vi "gyro-V5.vi"() -> ()   [LabVIEW 2017] (continued)
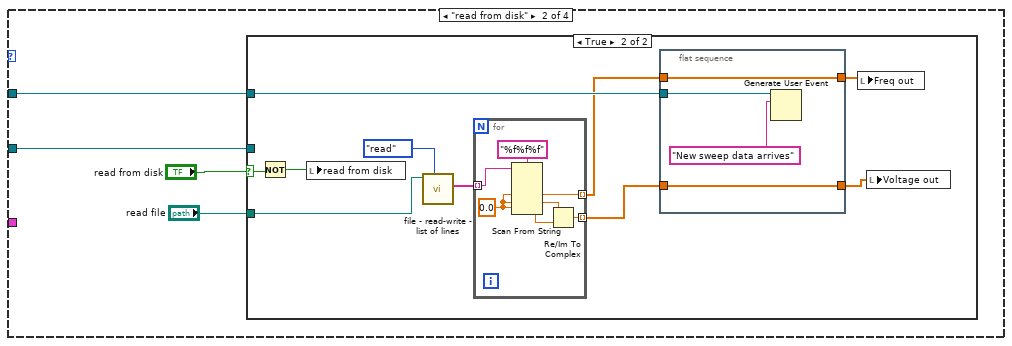
[diagram p4: hidden frame]
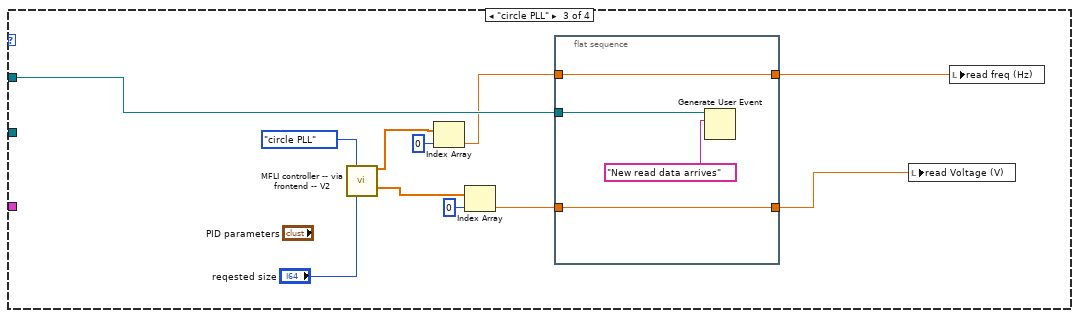
[diagram p6: hidden frame]
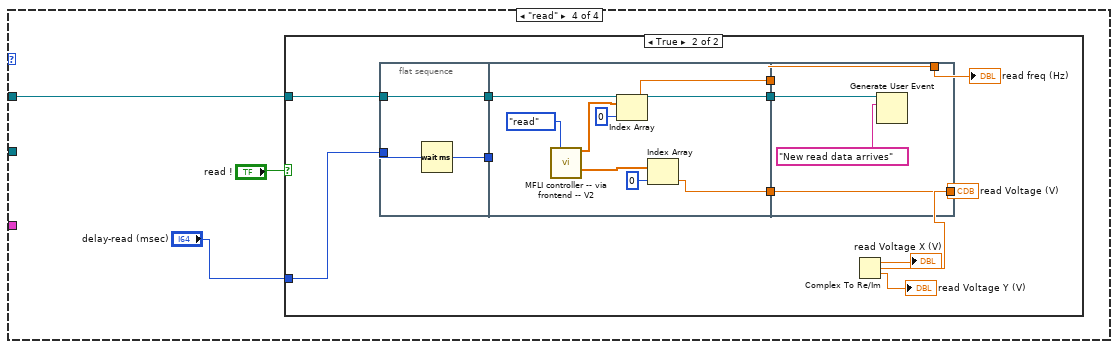
[diagram p7: hidden frame]
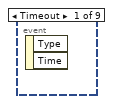
[diagram p9: hidden frame]
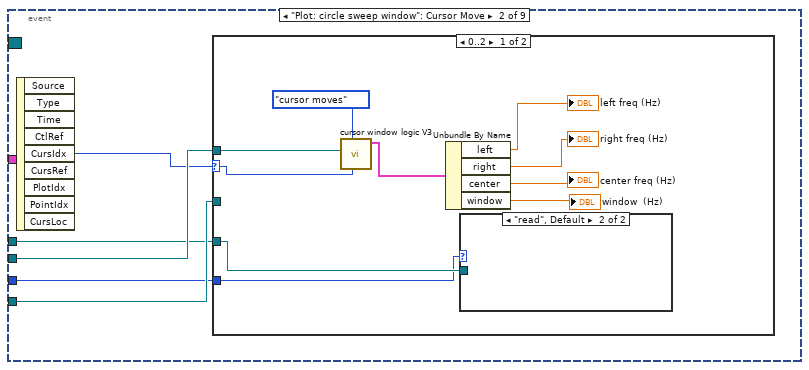
[diagram p10: hidden frame]
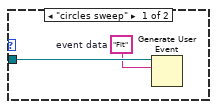
[diagram p11: hidden frame]
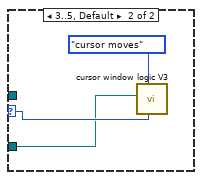
[diagram p12: hidden frame]
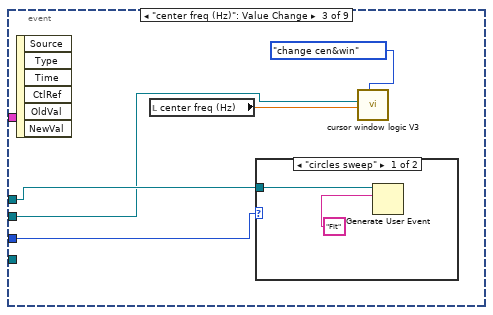
[diagram p13: hidden frame]
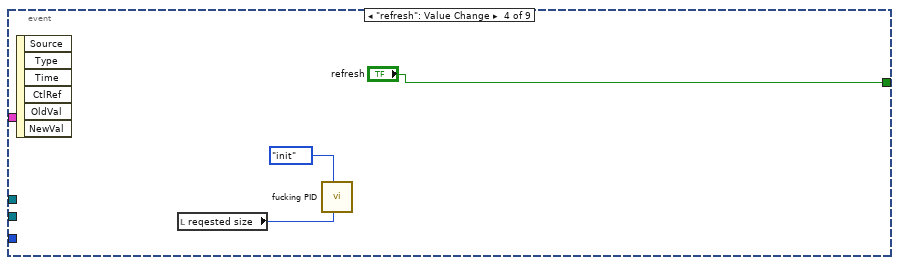
[diagram p15: hidden frame]
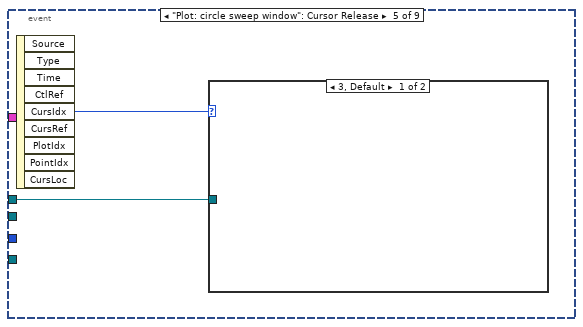
[diagram p16: hidden frame]
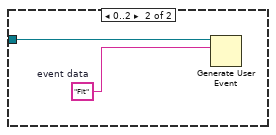
[diagram p17: hidden frame]
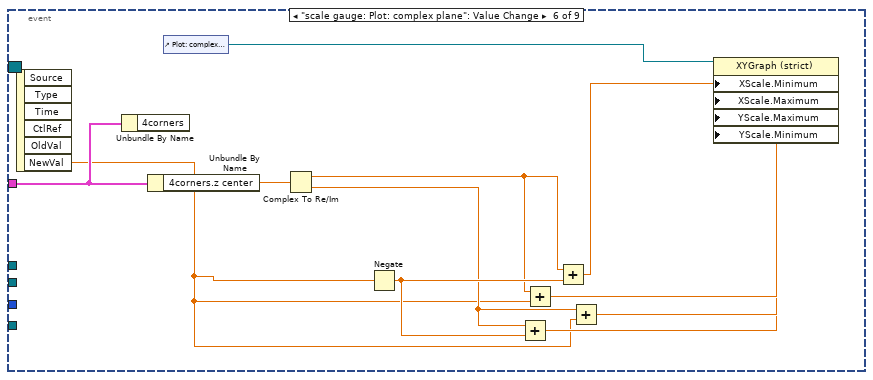
[diagram p18: hidden frame]
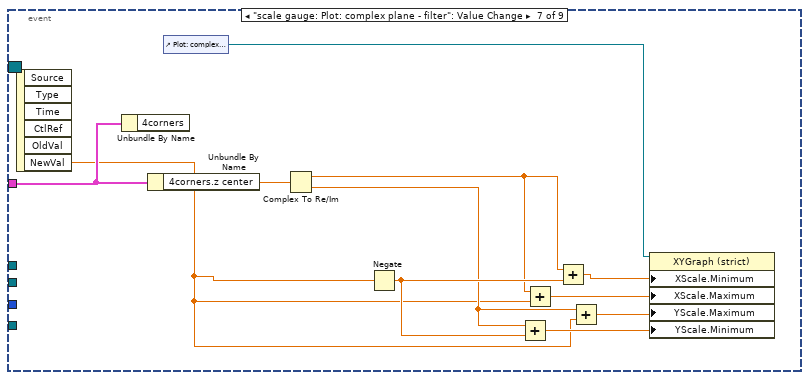
[diagram p19: hidden frame]
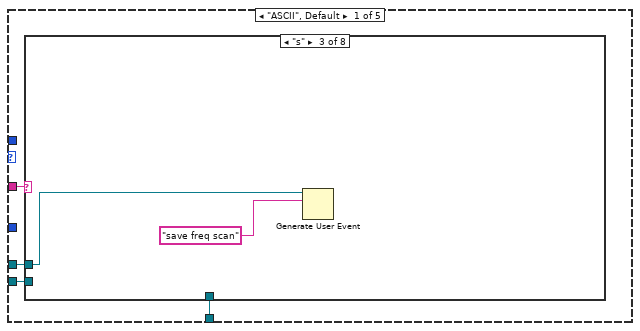
[diagram p20: hidden frame]
                  n39 = Re/Im To Complex(1:w95, 2:w96) -> (0:w94:cdb)
                }
                n40 = flat-sequence {
                  tunnel: w86 -> [w103]
                  tunnel: [w103] -> w85
                  tunnel: w92 -> [w102]
                  tunnel: [w101] -> w84
                  tunnel: w83 -> [w101]
                  frame #0 {
                    n41 = Generate User Event(user event=w102, event data cluster="New sweep data arrives" ("event data")) -> ()  [unwired: 2 in, 2 out]
                  }
                }
                n42 = local write "Freq out"(w85) -> ()
                n43 = local write "Voltage out"(w84) -> ()
              }
            }
          }
          frame "circle PLL" {
            n44 = call "MFLI controller -- via frontend -- V2.vi"("MFLI controller action"=MFLI_controller_action."circle PLL", "reqested size"="reqested size") -> ("Freq out (Hz)"=w111:dbl[], "Voltage out (V)"=w110:cdb[])  [unwired: 11 in, 1 out]
            n45 = Index Array(array=w111, index=0) -> (element=w107:dbl)
            n46 = Index Array(array=w110, index=0) -> (element=w105:cdb)
            n47 = flat-sequence {
              tunnel: w109 -> [w117]
              tunnel: [w116] -> w108
              tunnel: w107 -> [w116]
              tunnel: [w115] -> w106
              tunnel: w105 -> [w115]
              frame #0 {
                n48 = Generate User Event(user event=w117, event data cluster="New read data arrives" ("event data")) -> ()  [unwired: 2 in, 2 out]
              }
            }
            n49 = local write "read Voltage (V)"(w106) -> ()
            n50 = local write "read freq (Hz)"(w108) -> ()
          }
          frame "read" {
            n51 = case shown="True" "read !" {
              tunnel: w121 -> [_ w132]
              tunnel: "delay-read (msec)" -> [_ w126]
              frame False {
              }
              frame True {
                n52 = flat-sequence {
                  tunnel: w132 -> [w135]
                  tunnel: [w135] -> w127
                  tunnel: w126 -> [w134]
                  tunnel: [w133] -> w125
                  tunnel: [w136] -> w130
                  tunnel: [w143] -> w129
                  tunnel: [w137] -> w128
                  tunnel: w127 -> [w143]
                  tunnel: w125 -> [_]
                  tunnel: [w147] -> w131
                  tunnel: [w144] -> w124
                  tunnel: w130 -> [w147]
                  tunnel: w129 -> [w145]
                  tunnel: w128 -> [w144]
                  frame #0 {
                    n53 = Wait (ms)(milliseconds to wait=w134) -> (millisecond timer value=w133:u32)
                  }
                  frame #1 {
                    n54 = call "MFLI controller -- via frontend -- V2.vi"("MFLI controller action"=MFLI_controller_action."read") -> ("Freq out (Hz)"=w139:dbl[], "Voltage out (V)"=w141:cdb[])  [unwired: 12 in, 1 out]
                    n55 = Index Array(array=w139, index=0) -> (element=w136:dbl)
                    n56 = Index Array(array=w141, index=0) -> (element=w137:cdb)
                  }
                  frame #2 {
                    n57 = Generate User Event(user event=w145, event data cluster="New read data arrives" ("event data")) -> ()  [unwired: 2 in, 2 out]
                  }
                }
                n58 = Complex To Re/Im(x + iy=w124) -> (x=→"read Voltage X (V)":dbl, y=→"read Voltage Y (V)":dbl)
                "read freq (Hz)" <- w131
                "read Voltage (V)" <- w124
              }
            }
          }
        }
      }
    }
  }
  n59 = Create User Event(user event datatype=w38) -> (user event=w37:refnum<user-event>)  [unwired: 1 in, 1 out]
  n60 = register-events(w37) -> (reference out=w39:refnum<event-registration>)  [unwired: 2 in, 1 out]
  n61 = while {
    tunnel: w41 -> [w157]
    tunnel: w26 -> [w155]
    tunnel: w30 -> [w151]
    tunnel: w1 -> [w149]
    tunnel: w2 -> [w148]
    i -> [w152]
    stop <- FALSE stop-if-true
    n62 = Equal To 0?(x=w152) -> (x = 0?=w150:bool)
    n63 = event shown="[0] <calculate>: User Event" {
      selector: w157 -> [_ _]
      dyn-events: _ -> [_ _]
      timeout: 1 -> [_ _]
      tunnel: w155 -> [w165 _]
      tunnel: w151 -> [w162 _]
      tunnel: w150 -> [w161 _]
      tunnel: w149 -> [w160 _]
      tunnel: w148 -> [w158 _]
      event User Event {
        # "all z"
        # "all omega"
        n64 = event-data() -> ("calculate"=w166:string)  [unwired: 1 in]
        n65 = local read "pm lorentzian"() -> (w159:T8)
        n66 = for {
          N: 1 -> [_]
          tunnel: w166 -> [w178]
          tunnel: w165 -> [w177]
          shift-right: [w171] -> _
          shift-left: _ -> [w176]
          shift-right: [w170] -> _
          shift-left: _ -> [w175]
          tunnel: "Save folder" -> [w174]
          tunnel: w162 -> [w173]
          tunnel: w161 -> [w172]
          tunnel: w160 -> [w169]
          tunnel: w159 -> [w168]
          tunnel: w158 -> [w167]
          n67 = case shown="\"Fit\"" w178 {
            tunnel: w177 -> [w192 w248 _ _ _ _ _ _]
            tunnel: w176 -> [_ w247 w307 w326 w332 w354 w376 w419]
            tunnel: w175 -> [_ w246 w306 w325 w331 w353 w375 w418]
            tunnel: w174 -> [_ _ _ w321 w333 w351 _ _]
            tunnel: w173 -> [_ _ _ _ _ _ w378 _]
            tunnel: w172 -> [_ _ _ _ _ _ _ _]
            tunnel: [w183 w247 w307 w326 w332 w354 w376 w419] -> w171
            tunnel: [w181 w246 w306 w325 w331 w353 w375 w418] -> w170
            tunnel: w169 -> [_ _ _ _ _ w352 w377 _]
            tunnel: w168 -> [_ _ w292 w320 _ w350 _ _]
            tunnel: w167 -> [_ w245 _ _ _ w343 _ _]
            frame "New sweep data arrives" {
              n68 = local read "Voltage out"() -> (w182:cdb[])
              n69 = local read "Freq out"() -> (w184:dbl[])
              n70 = case shown="False" "subtract bgnd !" {
                tunnel: w184 -> [w204 w212]
                tunnel: [w198 w212] -> w183
                tunnel: w182 -> [w200 w211]
                tunnel: [w205 w211] -> w181
                frame True {
                  w197 = 10 ("length")
                  n71 = Delete From Array(array=w200, length=w197, index=0) -> (array with subset deleted=w199:cdb[])  [unwired: 1 out]
                  n72 = Delete From Array(array=w204, length=w197, index=0) -> (array with subset deleted=w203:dbl[])  [unwired: 1 out]
                  n73 = call "linear interp iiii- complex - z-omega.vi"("z"=w199, "omega"=w203) -> ("z out"=w206:cdb[], "omega out"=w198:dbl[], "intercept"=w208:cdb, "slope"=w209:cdb)  [unwired: 5 in, 5 out]
                  n74 = Multiply(x=w198, y=w209) -> (x*y=w210:cdb[])
                  n75 = Add(x=w210, y=w208) -> (x+y=w207:cdb[])
                  n76 = Subtract(x=w206, y=w207) -> (x-y=w205:cdb[])
                }
                frame False {
                }
              }
              n77 = Generate User Event(user event=w192, event data cluster="Fit" ("event data")) -> (user event out=w190:refnum<user-event>)  [unwired: 2 in, 1 out]
              n78 = case shown="True" "Auto-update sweep window!" {
                tunnel: w190 -> [w215 w217]
                tunnel: [w215 w216] -> w189
                frame False {
                }
                frame True {
                  n79 = Generate User Event(user event=w217, event data cluster="Update range" ("event data")) -> (user event out=w216:refnum<user-event>)  [unwired: 2 in, 1 out]
                }
              }
              n80 = Complex To Re/Im(x + iy=w181) -> (x=w195:dbl[], y=w194:dbl[])
              n81 = case shown="True" "Plot frequency shift" {
                tunnel: w189 -> [w219 w221]
                tunnel: [w219 w220] -> w186
                frame False {
                }
                frame True {
                  n82 = Generate User Event(user event=w221, event data cluster="Plot frequency shift" ("event data")) -> (user event out=w220:refnum<user-event>)  [unwired: 2 in, 1 out]
                }
              }
              n83 = Bundle("Freq out"=w183, w195) -> (w196:cluster{"Freq out":dbl[], dbl[]})  [unwired: 1 in]
              n84 = Bundle("Freq out"=w183, w194) -> (w193:cluster{"Freq out":dbl[], dbl[]})  [unwired: 1 in]
              n85 = case shown="True" "save data ?" {
                tunnel: w186 -> [_ w213]
                frame False {
                }
                frame True {
                  n86 = Generate User Event(user event=w213, event data cluster="save data" ("event data")) -> ()  [unwired: 2 in, 2 out]
                }
              }
              n87 = Build Array(w196, w193) -> (→"Plot: circle sweep window":cluster{"Freq out":dbl[], dbl[]}[])
            }
            frame "New read data arrives" {
              n88 = local read "read freq (Hz)"() -> (w224:dbl)
              n89 = local read "read Voltage (V)"() -> (w228:cdb)
              n90 = call "cursor window logic V3.vi"("cursor window action"=cursor_window_action."read", "cursor window in"=w245) -> ("cursor window out"=w243:T10)  [unwired: 8 in, 1 out]
              n91 = local read "pm lorentzian"() -> (w226:T8)
              n92 = Unbundle By Name(w243) -> ("Plot ref"=w242:refnum<vi>)
              n93 = call "replace cursor - plot ref - V2.vi"("Plot ref in"=w242, "new X"=w224, "cursor index"=6, "cursor action"=cursor_action."write") -> ()  [unwired: 13 in, 3 out]
              n94 = Bundle By Name(cluster=w226, "omega(0)"=w224) -> (w225:T8)
              n95 = local read "Plot frequency shift"() -> (w249:bool)
              n96 = for {
                N: 1 -> [_]
                shift-right: [w265] -> w239
                shift-left: _ -> [w264]
                tunnel: w228 -> [w263]
                tunnel: w224 -> [w262]
                shift-right: [w260] -> w237
                shift-left: _ -> [w261]
                tunnel: "aggregator action" -> [w258]
                w259 = 10000
                n97 = call "aggregator - vii - real - atomic.vi"("aggregator action"=w258, "requested size"=w259, "number"=w262, "state IN"=w261) -> ("state OUT"=w260:T26)  [unwired: 4 in, 3 out]
                n98 = call "aggregator - vii - complex - atomic.vi"("aggregator action"=w258, "requested size"=w259, "number"=w263, "state IN"=w264) -> ("state OUT"=w265:T27)  [unwired: 4 in, 3 out]
              }
              n99 = case shown="True" w249 {
                tunnel: w248 -> [w268 w270]
                tunnel: [w268 w269] -> w251
                frame False {
                }
                frame True {
                  n100 = Generate User Event(user event=w270, event data cluster="Plot frequency shift" ("event data")) -> (user event out=w269:refnum<user-event>)  [unwired: 2 in, 1 out]
                }
              }
              n101 = local write "pm lorentzian"(w225) -> ()
              n102 = Unbundle By Name(w237) -> ("Array"=w235:dbl[])
              n103 = local read "save data ?"() -> (w250:bool)
              n104 = Unbundle By Name(w239) -> ("Array"=w232:cdb[])
              n105 = Complex To Re/Im(x + iy=w232) -> (x=w231:dbl[], y=w230:dbl[])
              n106 = Bundle(w231, w230) -> (→"Plot: frequency shift vs T 4":cluster{dbl[], dbl[]})  [unwired: 1 in]
              n107 = Array Size(array=w235) -> (size(s)=w236:i32)
              n108 = case shown="True" w250 {
                tunnel: w251 -> [_ w266]
                frame False {
                }
                frame True {
                  n109 = Generate User Event(user event=w266, event data cluster="save data" ("event data")) -> ()  [unwired: 2 in, 2 out]
                }
              }
              n110 = for {
                N: w236 -> [_]
                tunnel: [w257] -> w234 mode=indexing
                i -> [w257]
              }
              n111 = Bundle(w234, "Array"=w235) -> (→"Plot: frequency shift vs T 5":cluster{i32[], "Array":dbl[]})  [unwired: 1 in]
              n112 = case shown="\"save\", Default" "save number to dropbox" {
                tunnel: w224 -> [w256 _]
                frame "save", Default {
                  n113 = call "KM_appendline --readfreq.vi"("freq"=w256, "append to file? (new file:F)"=FALSE, "Save frequency scan"="Save read folder", "read/write control"=KM_file_--_read-write_control."append one line", "name or relative path"="read file name") -> ()  [unwired: 15 in]
                }
                frame "do not save" {
                }
              }
            }
            frame "Plot frequency shift" {
              (unwired) T4."background"
              (unwired) enum16{"Time", "temperature", "field", "angle"}."angle"
              w274 = 1000000 ("requested size")
              # "omega (Hz)"
              # "time (min)"
              n114 = Unbundle By Name(w292) -> ("omega(0)"=w297:dbl, "Gamma"=w296:dbl, "phase"=w278:dbl, "z (inf)"=w276:cdb)
              n115 = call <vilib>:"High Resolution Relative Seconds.vi"() -> ("relative seconds"=w298:dbl)
              n116 = Divide(x=w298, y=60) -> (x/y=w300:dbl)
              n117 = Complex To Polar(r * e^(i*theta)=w276) -> (r=w275:dbl)  [unwired: 1 out]
              n118 = Multiply(x="plot length (min)", y=60) -> (x*y=w302:dbl)
              n119 = call "fancy torque read T .vi"() -> ("angle"=w284:dbl, "field"=w285:dbl, "temperature"=w291:dbl)  [unwired: 8 in, 1 out]
              n120 = Divide(x=w302, y="aggregate every # sec") -> (x/y=w301:dbl)
              n121 = Round Toward +Infinity(x=w301) -> (ceil(x): smallest int >= x=w304:dbl)
              n122 = call "switch - C.vi"("switch"=TRUE) -> ("result"=w272:bool)  [unwired: 10 in]
              n123 = To Long Integer(number=w304) -> ()  [unwired: 1 out]
              n124 = call "aggregator - v - real.vi"("number"=w275, "init?"=w272, "requested size"=w274) -> ("Array"=w273:dbl[])  [unwired: 6 in, 2 out]
              n125 = call "aggregator - v - real.vi"("number"=w278, "init?"=w272, "requested size"=w274) -> ("Array"=w277:dbl[])  [unwired: 6 in, 2 out]
              n126 = call "aggregator - v - real.vi"("number"=w300, "init?"=w272, "requested size"=w274) -> ("Array"=w287:dbl[])  [unwired: 6 in, 2 out]
              n127 = call "aggregator - v - real.vi"("number"=w297, "init?"=w272, "requested size"=w274) -> ("Array"=w280:dbl[])  [unwired: 6 in, 2 out]
              n128 = call "aggregator - v - real.vi"("number"=w296, "init?"=w272, "requested size"=w274) -> ("Array"=w279:dbl[])  [unwired: 6 in, 2 out]
              n129 = call "aggregator - v - real.vi"("number"=w291, "init?"=w272, "requested size"=w274) -> ("Array"=w289:dbl[])  [unwired: 6 in, 2 out]
              n130 = call "aggregator - v - real.vi"("number"=w285, "init?"=w272, "requested size"=w274) -> ("Array"=w286:dbl[])  [unwired: 6 in, 2 out]
              n131 = call "aggregator - v - real.vi"("number"=w284, "init?"=w272, "requested size"=w274) -> ("Array"=w283:dbl[])  [unwired: 6 in, 2 out]
              n132 = case shown="\"angle\"" "horisontal axis" {
                tunnel: w289 -> [_ w313 _ _]
                tunnel: [w312 w313 w314 w315] -> w288
                tunnel: w287 -> [w312 _ _ _]
                tunnel: w286 -> [_ _ w314 _]
                tunnel: w283 -> [_ _ _ w315]
                frame "Time", Default {
                }
                frame "temperature" {
                }
                frame "field" {
                }
                frame "angle" {
                }
              }
              n133 = case shown="\"gamma\"" "vertical axis" {
                tunnel: w279 -> [_ w309 _ _]
                tunnel: [w308 w309 w310 w311] -> w281
                tunnel: w280 -> [w308 _ _ _]
                tunnel: w277 -> [_ _ w310 _]
                tunnel: w273 -> [_ _ _ w311]
                frame "frequency", Default {
                }
                frame "gamma" {
                }
                frame "phase" {
                }
                frame "background" {
                }
              }
              n134 = Bundle("Array"=w288, "Array"=w281) -> (→"Plot: frequency shift vs T":cluster{"Array":dbl[], "Array":dbl[]})  [unwired: 1 in]
            }
            frame "save data" {
              n135 = call <vilib>:"High Resolution Relative Seconds.vi"() -> ("relative seconds"=w319:dbl)
              n136 = call "fancy torque read T .vi"() -> ("angle"=w316:dbl, "field"=w318:dbl, "temperature"=w317:dbl)  [unwired: 8 in, 1 out]
              "Field (T)" <- w318
              "Temperature (K)" <- w317
              "angle (deg)" <- w316
              n137 = call "switch - C.vi"("switch"=TRUE) -> ()  [unwired: 10 in, 1 out]
              n138 = call "KM_appendline.vi"("Time (s)"=w319, "temperature"=w317, "Field"=w318, "angle (deg)"=w316, "pm lorentzian"=w320, "Save frequency scan"=w321, "read/write control"=KM_file_--_read-write_control."append one line", "name or relative path"="data file name") -> ()  [unwired: 12 in]
            }
            frame "save freq scan" {
              n139 = local read "freqsweep pattern"() -> (w328:T3)
              n140 = call "filename-manage.vi"("filename pattern"=w328, "filename-action"=filename-action."parse", "file name"="freq sweep file name") -> ("filename OUT"=w327:string)  [unwired: 8 in]
              n141 = local write "freq sweep file name"(w327) -> ()
              n142 = call "KM_appendline -- freq sweep.vi"("freq"=w332, "Vout(V)"=w331, "Save frequency scan"=w333, "read/write control"=KM_file_--_read-write_control."append one line", "name or relative path"=w327) -> ()  [unwired: 15 in]
            }
            frame "Update range" {
              n143 = Unbundle By Name(w350) -> ("omega(0)"=w341:dbl, "Gamma"=w348:dbl)
              n144 = call "cursor window logic V3.vi"("cursor window action"=cursor_window_action."read", "cursor window in"=w343) -> ("cursor window out"=w346:T10)  [unwired: 8 in, 1 out]
              n145 = Unbundle By Name(w346) -> ("left"=w345:dbl, "right"=w344:dbl, "window"=w338:dbl)
              n146 = Multiply(x=w338, y=3.0 ("lower")) -> (x*y=w339:dbl)
              n147 = Multiply(x=w338, y=0.0003 ("lower")) -> (x*y=w336:dbl)
              n148 = call "Q -- check range -- i -- real.vi"("upper"=w344, "lower"=w345, "number"=w341) -> ("in range?"=w349:bool)  [unwired: 6 in, 2 out]
              n149 = call "Q -- check range -- i -- real.vi"("upper"=w339, "lower"=w336, "number"=w348) -> ("in range?"=w347:bool)  [unwired: 6 in, 2 out]
              n150 = And(x=w349, y=w347) -> (x .and. y?=w342:bool)
              "fit is fine" <- w342
              n151 = case shown="True" w342 {
                tunnel: w348 -> [_ w362]
                tunnel: w341 -> [_ w356]
                tunnel: w352 -> [_ w363]
                tunnel: w351 -> [_ _]
                frame False {
                }
                frame True {
                  (unwired) agregator_--_action."append" ("aggregator action")
                  n152 = Compound Arithmetic op=MULTIPLY("gamma factor", w362, 2.0 ("value")) -> (w360:dbl)
                  n153 = for {
                    N: 1 -> [_]
                    tunnel: "history length" -> [w367]
                    tunnel: w356 -> [w372]
                    shift-right: [w368] -> _
                    shift-left: _ -> [w371]
                    tunnel: [w365] -> w355
                    n154 = call "aggregator - vii - real - atomic.vi"("aggregator action"=agregator_--_action."append", "requested size"=w367, "number"=w372, "state IN"=w371) -> ("state OUT"=w369:T26)  [unwired: 4 in, 3 out]
                    n155 = call "aggregator - vii - real - atomic.vi"("aggregator action"=agregator_--_action."interpolate", "requested size"=w367, "state IN"=w369) -> ("interp average"=w365:dbl, "state OUT"=w368:T26)  [unwired: 5 in, 2 out]
                  }
                  n156 = call "cursor window logic V3.vi"("cursor window action"=cursor_window_action."change cen&win", "window"=w360, "center"=w355, "cursor window in"=w363) -> ()  [unwired: 6 in, 2 out]
                }
              }
            }
            frame "Fit" {
              n157 = case shown="True" "fit?" {
                tunnel: w378 -> [_ w395]
                tunnel: w377 -> [_ w393]
                tunnel: w376 -> [_ w391]
                tunnel: w375 -> [_ w388]
                tunnel: [T8 {"Amplitude"=-1.0311345636926572, "omega(0)"=-1.0311345636926572, "Gamma"=-1.0311345636926572, "phase"=-1.0311345636926572, "Q"=-1.0311345636926572, "Norm  Ampl"=-1.0311345636926572, "z (inf)"=-1.0311345636926572+0.0i, "4corners"={"z (-pi/2)"=-1.0311345636926572+0.5736824521422934i, "z(inf)"=-0.5200164984937075+1.0975277942502903i, "z (pi/2)"=-1.0311345636926572+0.5736824521422934i, "z center"=-0.5136528600391839+0.580046090596817i, "z(0)"=-0.5200164984937075+1.0975277942502903i, "radius"=-1.0311345636926572}} ("pm lorentzian") w380] -> w374
                frame False {
                }
                frame True {
                  n158 = call "cursor window logic V3.vi"("cursor window action"=cursor_window_action."read", "cursor window in"=w393) -> ("cursor window out"=w389:T10)  [unwired: 8 in, 1 out]
                  n159 = Increment(x="some") -> (x+1=w382:dbl)
                  n160 = local write "some"(w382) -> ()
                  n161 = call "acquire cursor window data.vi"("z in"=w388, "omega in"=w391, "cursor window"=w389) -> ("z out"=w390:cdb[], "omega  out"=w392:dbl[])  [unwired: 4 in, 3 out]
                  n162 = call "KM_peak -- find -- pm - V1.vi"("omega in"=w392, "z in"=w390, "parameters: complex fit"="parameters: complex fit", "plots: filter related"=w395, "plot staff ?"="plot staff", "just guess?"="use fast fit?", "subtract linear BG"=FALSE) -> ("pm lorentzian"=w380:T8)  [unwired: 10 in, 2 out]
                  n163 = local write "pm lorentzian"(w380) -> ()
                  n164 = Unbundle By Name(w380) -> ("omega(0)"=→"circle frequency (Hz)":dbl, "Gamma"=→"circle gamma (Hz)":dbl, "phase"=→"circle phase (rad)":dbl, "Q"=→"circle Q":dbl)
                  n165 = call "MFLI -- publish -- fake lever lor.vi"("publisher action"=publisher_action."set", "lorentzian IN"=w380) -> ()  [unwired: 9 in, 1 out]
                }
              }
              n166 = disable-structure shown="Disabled" {
                disable-tunnel: w374 -> [w408 _]
                disable-tunnel: w375 -> [w407 _]
                frame Disabled {
                  n167 = for {
                    tunnel: four-corner_circle_transformation."to  canonical" ("4 corner circle transformation") -> [w417]
                    tunnel: w408 -> [w416]
                    tunnel: w407 -> [w415] mode=indexing
                    tunnel: [w414] -> w406 mode=indexing
                    n168 = call "lorentzian transformations.vi"("4 corner circle transformation"=w417, "lorentzian in"=w416, "voltage in"=w415) -> ("voltage out"=w414:cdb)  [unwired: 6 in, 2 out]
                  }
                  n169 = Complex To Polar(r * e^(i*theta)=w406) -> (theta=w404:dbl[])  [unwired: 1 out]
                  n170 = Complex To Re/Im(x + iy=w406) -> (x=w411:dbl[], y=w412:dbl[])
                  n171 = Bundle(w411, w412) -> (→"Plot: frequency shift vs T 2":cluster{dbl[], dbl[]})  [unwired: 1 in]
                  n172 = Add(x=w404, y=1.5707963267948966) -> (x+y=w402:dbl[])
                  n173 = Array Size(array=w402) -> (size(s)=w403:i32)
                  n174 = for {
                    N: w403 -> [_]
                    tunnel: [w413] -> w401 mode=indexing
                    i -> [w413]
                  }
                  n175 = Bundle(w401, w402) -> (→"Plot: frequency shift vs T 3":cluster{i32[], dbl[]})  [unwired: 1 in]
                }
                frame Enabled {
                }
              }
            }
            frame "Void", Default {
            }
          }
        }
      }
      event Timeout {
        n176 = event-data() -> ()  [unwired: 1 in, 2 out]
      }
    }
    n177 = Wait (ms)(milliseconds to wait=u32 0) -> ()  [unwired: 1 out]
  }
  n178 = while {
    tunnel: w39 -> [w427]
    tunnel: w26 -> [w425]
    tunnel: w1 -> [w424]
    tunnel: w2 -> [w421]
    stop <- FALSE stop-if-true
    n179 = local read "pm lorentzian"() -> (w423:T8)
    n180 = local read "MFLI mode"() -> (w420:T1)
    n181 = event shown="[7] Key Down" {
      selector: w427 -> [_ _ _ _ _ _ _ _ _]
      dyn-events: _ -> [_ _ _ _ _ _ _ _ _]
      timeout: _ -> [_ _ _ _ _ _ _ _ _]
      tunnel: w425 -> [_ w429 w450 _ w459 _ _ w490 w548]
      tunnel: [_ _ _ _ _ _ _ _ "Update system parameters"] -> _
      tunnel: w424 -> [_ w432 w449 _ _ _ _ w486 _]
      tunnel: w423 -> [_ _ _ _ _ w464 w475 _ _]
      tunnel: w421 -> [_ w430 _ _ _ _ _ w485 _]
      tunnel: [_ _ _ "refresh" _ _ _ _ _] -> _
      tunnel: w420 -> [_ w428 w448 _ _ _ _ _ _]
      event Timeout {
        n182 = event-data() -> ()  [unwired: 1 in, 2 out]
      }
      event "Plot: circle sweep window": Cursor Move {
        n183 = event-data() -> ("CursIdx"=w431:i32)  [unwired: 1 in, 8 out]
        n184 = case shown="0..2" w431 {
          selector: w431 -> [w440 w446]
          tunnel: w432 -> [w442 _]
          tunnel: w430 -> [_ w445]
          tunnel: w429 -> [w434 _]
          tunnel: w428 -> [w433 _]
          frame 0..2 {
            n185 = call "cursor window logic V3.vi"("CursIdx"=w440, "cursor window action"=cursor_window_action."cursor moves", "cursor window in"=w442) -> ("cursor window out"=w439:T10)  [unwired: 7 in, 1 out]
            n186 = Unbundle By Name(w439) -> ("left"=→"left freq (Hz)":dbl, "right"=→"right freq (Hz)":dbl, "center"=→"center freq (Hz)":dbl, "window"=→"window  (Hz)":dbl)
            n187 = case shown="\"read\", Default" w433 {
              tunnel: w434 -> [w444 _]
              frame "circles sweep" {
                w443 = "Fit"  # event data
                n188 = Generate User Event(user event=w444, event data cluster=w443) -> ()  [unwired: 2 in, 2 out]
              }
              frame "read", Default {
              }
            }
          }
          frame 3..5, Default {
            n189 = call "cursor window logic V3.vi"("CursIdx"=w446, "cursor window action"=cursor_window_action."cursor moves", "cursor window in"=w445) -> ()  [unwired: 7 in, 2 out]
          }
        }
      }
      event "center freq (Hz)": Value Change {
        n190 = event-data() -> ()  [unwired: 1 in, 6 out]
        n191 = local read "center freq (Hz)"() -> (w451:dbl)
        n192 = case shown="\"circles sweep\"" w448 {
          tunnel: w450 -> [w454 _]
          frame "circles sweep" {
            n193 = Generate User Event(user event=w454, event data cluster="Fit" ("event data")) -> ()  [unwired: 2 in, 2 out]
          }
          frame "read", Default {
          }
        }
        n194 = call "cursor window logic V3.vi"("cursor window action"=cursor_window_action."change cen&win", "center"=w451, "cursor window in"=w449) -> ()  [unwired: 7 in, 2 out]
      }
      event "refresh": Value Change {
        n195 = event-data() -> ()  [unwired: 1 in, 6 out]
        n196 = local read "reqested size"() -> (w455:i64)
        n197 = call "fucking PID.vi"("requested size"=w455, "PID action"=agregator_--_action."init") -> ()  [unwired: 6 in, 4 out]
      }
      event "Plot: circle sweep window": Cursor Release {
        n198 = event-data() -> ("CursIdx"=w458:i32)  [unwired: 1 in, 8 out]
        n199 = case shown="3, Default" w458 {
          tunnel: w459 -> [_ w460]
          frame 3, Default {
          }
          frame 0..2 {
            w461 = "Fit"  # event data
            n200 = Generate User Event(user event=w460, event data cluster=w461) -> ()  [unwired: 2 in, 2 out]
          }
        }
      }
      event "scale gauge: Plot: complex plane": Value Change {
        n201 = event-data() -> ("NewVal"=w463:dbl)  [unwired: 1 in, 5 out]
        n202 = Unbundle By Name(w464) -> ()  [unwired: 1 out]
        n203 = Unbundle By Name(w464) -> ("4corners.z center"=w465:cdb)
        n204 = control-ref of="Plot: complex plane"() -> (w462:refnum<vi>)
        n205 = Complex To Re/Im(x + iy=w465) -> (x=w466:dbl, y=w467:dbl)
        n206 = Negate(x=w463) -> (-x=w472:dbl)
        n207 = Add(x=w467, y=w472) -> (x+y=w468:dbl)
        n208 = Add(x=w466, y=w463) -> (x+y=w470:dbl)
        n209 = Add(x=w466, y=w472) -> (x+y=w471:dbl)
        n210 = Add(x=w467, y=w463) -> (x+y=w469:dbl)
        n211 = property on="Property Node" class="XYGraph (strict)"(reference=w462, "XScale.Minimum"=w471, "XScale.Maximum"=w470, "YScale.Maximum"=w469, "YScale.Minimum"=w468) -> ()  [unwired: 1 in, 2 out]
      }
      event "scale gauge: Plot: complex plane - filter": Value Change {
        n212 = event-data() -> ("NewVal"=w474:dbl)  [unwired: 1 in, 5 out]
        n213 = Unbundle By Name(w475) -> ()  [unwired: 1 out]
        n214 = Unbundle By Name(w475) -> ("4corners.z center"=w476:cdb)
        n215 = control-ref of="Plot: complex plane - filter"() -> (w473:refnum<vi>)
        n216 = Complex To Re/Im(x + iy=w476) -> (x=w477:dbl, y=w478:dbl)
        n217 = Negate(x=w474) -> (-x=w483:dbl)
        n218 = Add(x=w478, y=w483) -> (x+y=w479:dbl)
        n219 = Add(x=w477, y=w474) -> (x+y=w481:dbl)
        n220 = Add(x=w477, y=w483) -> (x+y=w482:dbl)
        n221 = Add(x=w478, y=w474) -> (x+y=w480:dbl)
        n222 = property on="Property Node" class="XYGraph (strict)"(reference=w473, "XScale.Minimum"=w482, "XScale.Maximum"=w481, "YScale.Maximum"=w480, "YScale.Minimum"=w479) -> ()  [unwired: 1 in, 2 out]
      }
      event Key Down {
        n223 = event-data() -> ("Char"=w488:i16, "VKey"=w491:T15)  [unwired: 1 in]
        "Char" <- w488
        "VKey" <- w491
        n224 = local read "MFLI mode"() -> (w484:T1)
        n225 = Build Array(w488) -> (w489:i16[])
        n226 = Byte Array To String(unsigned byte array=w489) -> (string=w487:string)
        n227 = case shown="\"Up\"..\"Right\"" w491 {
          selector: w491 -> [_ _ _ _ w539]
          tunnel: w488 -> [_ _ _ _ _]
          tunnel: w490 -> [w495 _ _ _ w538]
          tunnel: w487 -> [w494 _ _ _ _]
          tunnel: w486 -> [w493 _ _ _ w531]
          tunnel: w485 -> [w492 _ _ _ _]
          tunnel: w484 -> [_ _ _ _ w530]
          frame "ASCII", Default {
            n228 = case shown="\"s\"" w494 {
              selector: w494 -> [_ _ _ _ w503 _ _ _]
              tunnel: w495 -> [_ _ w498 _ _ _ _ _]
              tunnel: w493 -> [_ w496 _ w500 w504 w511 w514 w529]
              tunnel: w492 -> [_ _ _ _ _ w509 _ _]
              frame "0", Default {
              }
              frame "a" {
                n229 = call "cursor window logic V3.vi"("cursor window action"=cursor_window_action."zoom to all data", "cursor window in"=w496) -> ()  [unwired: 8 in, 2 out]
              }
              frame "s" {
                n230 = Generate User Event(user event=w498, event data cluster="save freq scan" ("event data")) -> ()  [unwired: 2 in, 2 out]
              }
              frame "?" {
                # "?"
                n231 = call "cursor window logic V3.vi"("cursor window action"=cursor_window_action."zoom X", "cursor window in"=w500) -> ()  [unwired: 8 in, 2 out]
              }
              frame "+", "-", "<", ">" {
                # "?"
                n232 = case shown="\"+\", Default" w503 {
                  tunnel: [cursor_window_action."slide right" ("cursor window action") cursor_window_action."slide left" ("cursor window action") cursor_window_action."zoom in" ("cursor window action") cursor_window_action."zoom out" ("cursor window action")] -> w502
                  frame ">" {
                  }
                  frame "<" {
                  }
                  frame "+", Default {
                  }
                  frame "-" {
                  }
                }
                n233 = call "cursor window logic V3.vi"("cursor window action"=w502, "cursor window in"=w504) -> ()  [unwired: 8 in, 2 out]
              }
              frame "c" {
                n234 = call "cursor window logic V3.vi"("cursor window action"=cursor_window_action."check", "cursor window in"=w511) -> ()  [unwired: 8 in, 2 out]
                n235 = call "cursor window logic V3.vi"("cursor window action"=cursor_window_action."check", "cursor window in"=w509) -> ()  [unwired: 8 in, 2 out]
              }
              frame "t" {
                n236 = local read "talk to MFLI !"() -> (w513:bool)
                n237 = case shown="True" w513 {
                  tunnel: w514 -> [_ w520]
                  frame False {
                  }
                  frame True {
                    n238 = local read "Auto-update sweep window!"() -> (w519:bool)
                    n239 = Not(x=w519) -> (.not. x?=w518:bool)
                    n240 = local write "Auto-update sweep window!"(w518) -> ()
                    n241 = Select(t=cursor_window_action."color--green" ("cursor window action"), s=w518, f=cursor_window_action."color--red" ("cursor window action")) -> (s? t:f=w515:T16)
                    n242 = call "cursor window logic V3.vi"("cursor window action"=w515, "cursor window in"=w520) -> ()  [unwired: 8 in, 2 out]
                  }
                }
              }
              frame "r" {
                n243 = local read "Auto-update sweep window!"() -> (w524:bool)
                n244 = local read "talk to MFLI !"() -> (w525:bool)
                n245 = Not(x=w525) -> (.not. x?=w528:bool)
                n246 = Select(t=cursor_window_action."color--green" ("cursor window action"), s=w524, f=cursor_window_action."color--red" ("cursor window action")) -> (s? t:f=w521:T16)
                n247 = Select(t=w521, s=w528, f=cursor_window_action."color--yellow" ("cursor window action")) -> (s? t:f=w526:T16)
                n248 = local write "talk to MFLI !"(w528) -> ()
                n249 = call "cursor window logic V3.vi"("cursor window action"=w526, "cursor window in"=w529) -> ()  [unwired: 8 in, 2 out]
              }
            }
          }
          frame "Escape" {
          }
          frame "PageUp" {
          }
          frame "PageDown" {
          }
          frame "Up".."Right" {
            n250 = case shown="\"Left\"" w539 {
              tunnel: [cursor_window_action."move right" ("cursor window action") cursor_window_action."move left" ("cursor window action") cursor_window_action."broaden" ("cursor window action") cursor_window_action."shrink" ("cursor window action")] -> w533
              frame "Right", Default {
              }
              frame "Left" {
              }
              frame "Up" {
              }
              frame "Down" {
              }
            }
            n251 = call "cursor window logic V3.vi"("cursor window action"=w533, "cursor window in"=w531) -> ("cursor window out"=w532:T10)  [unwired: 8 in, 1 out]
            n252 = Unbundle By Name(w532) -> ("left"=w537:dbl, "right"=w536:dbl, "center"=w535:dbl, "window"=w534:dbl)
            n253 = case shown="\"read from disk\"" w530 {
              tunnel: w538 -> [w541 w543 _]
              frame "circles sweep" {
                w540 = "Fit"  # event data
                n254 = Generate User Event(user event=w541, event data cluster=w540) -> ()  [unwired: 2 in, 2 out]
              }
              frame "read from disk" {
                w542 = "Fit"  # event data
                n255 = Generate User Event(user event=w543, event data cluster=w542) -> ()  [unwired: 2 in, 2 out]
              }
              frame "read", Default {
              }
            }
            n256 = local write "window  (Hz)"(w534) -> ()
            n257 = local write "right freq (Hz)"(w536) -> ()
            n258 = local write "center freq (Hz)"(w535) -> ()
            n259 = local write "left freq (Hz)"(w537) -> ()
          }
        }
      }
      event "Update system parameters": Value Change {
        n260 = event-data() -> ()  [unwired: 1 in, 6 out]
        n261 = Generate User Event(user event=w548, event data cluster="Update system parameters" ("event data")) -> ()  [unwired: 2 in, 2 out]
      }
    }
    n262 = Wait (ms)(milliseconds to wait=u32 0) -> ()  [unwired: 1 out]
  }
